vi "ADIS16448 IMU Example.vi"() -> ()   [LabVIEW 2018]
doc: "SimpleGyro Example\n\nThis example shows how to use a SimpleGyro sensor connected to the SPI port on the RoboRIO.\n\nThis example expects a USB cable connected from your development PC to the Type B USB Jack (next to the power input) on the roboRIO."
uses:
  ADIS16448 IMU/ADIS16448_IMU.lvlib
panel:
  out "Number of times failed":i32
  in  "Stahp":bool
  out "error out":errorcluster
  out "Z Angle":dbl
  in  "Calibrate On Open?":bool=TRUE
  out "IMU Angle Delta":cluster{"X":dbl, "Y":dbl, "Z":dbl} {"X" scale=-180.0..180.0; "Y" scale=-180.0..180.0; "Z" scale=-180.0..180.0}
  out "IMU AHRS":cluster{"Pitch":dbl, "Roll":dbl, "Yaw":dbl} {"Roll" scale=-180.0..180.0; "Pitch" scale=-90.0..90.0}
  out "IMU Data Out":T1 {"X Accel (g)" format="%#_3g"; "Y Accel (g)" format="%#_3g"; "Z Accel (g)" format="%#_3g"}
  in  "AHRS Algorithm":enum16{"Complementary", "Madgwick"}(ring)
  in  "AHRS Yaw Axis":enum16{"X", "Y", "Z"}(ring)=enum."Z"
  out "Sensor Ready?":bool
  out "IMU AHRS":cluster{"Pitch":dbl, "Roll":dbl, "Yaw":dbl}
  out "IMU Angle Delta":cluster{"X":dbl, "Y":dbl, "Z":dbl}
  in  "Reset Deltas?":bool
  out "Device Found?":bool
  in  "stop":bool
  # "FRC Analog Devices ADIS16448 IMU Example"
  # "Raw IMU Output Data"
  # "FRC ADI MXP Placement"
  # "Minimum LabVIEW version required: FRC 2019.0.0"
  # "Juan Chong -  Analog Devices Inc. - juan.chong@analog.com"
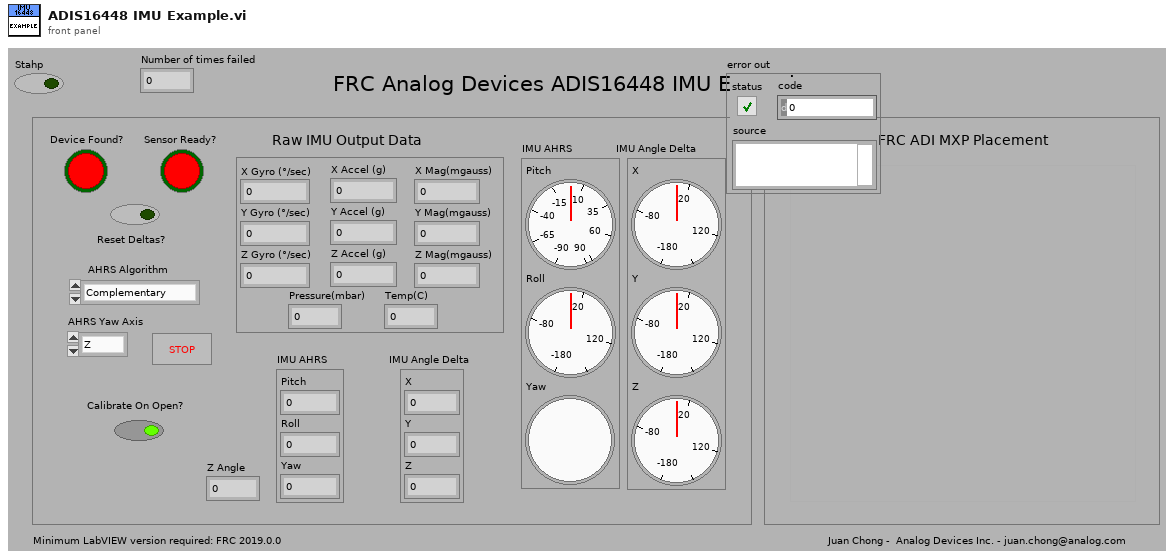
[diagram p1: front panel]
types:
  T1 = cluster{"X Gyro (°/sec)":dbl, "Y Gyro (°/sec)":dbl, "Z Gyro (°/sec)":dbl, "X Accel (g)":dbl, "Y Accel (g)":dbl, "Z Accel (g)":dbl, "X Mag(mgauss)":dbl, "Y Mag(mgauss)":dbl, "Z Mag(mgauss)":dbl, "Pressure(mbar)":dbl, "Temp(C)":dbl}
  T2 = typedef "ADIS16448_IMU.lvlib/ADI_IMU_ADIS16448_IMUDevRef.ctl" = cluster{"DevStatus":errorcluster, "Handle":i32, "SPI Bus":T3, "Device Found":bool, "Device Ready":bool, "Yaw Axis":enum16{"X", "Y", "Z"}, "AHRS Algorithm":enum16{"Complementary", "Madgwick"}, "Serial":u16, "Lot ID 2":u16, "Lot ID 1":u16, "Bytes Per Sample":u16, "Calibrate On Open?":bool}
  T3 = typedef "spi_bus.ctl" = enum16{"SPI On-Board, CS0", "SPI On-Board, CS1", "SPI On-Board, CS2", "SPI On-Board, CS3", "SPI MXP", "Invalid"}
  T4 = cluster{"X Angle":dbl, "Y Angle":dbl, "Z Angle":dbl}
  T5 = cluster{"X Gyro":dbl, "Y Gyro":dbl, "Z Gyro":dbl, "X Accel":dbl, "Y Accel":dbl, "Z Accel":dbl, "X Mag":dbl, "Y Mag":dbl, "Z Mag":dbl, "Pressure":dbl, "Temp":dbl}
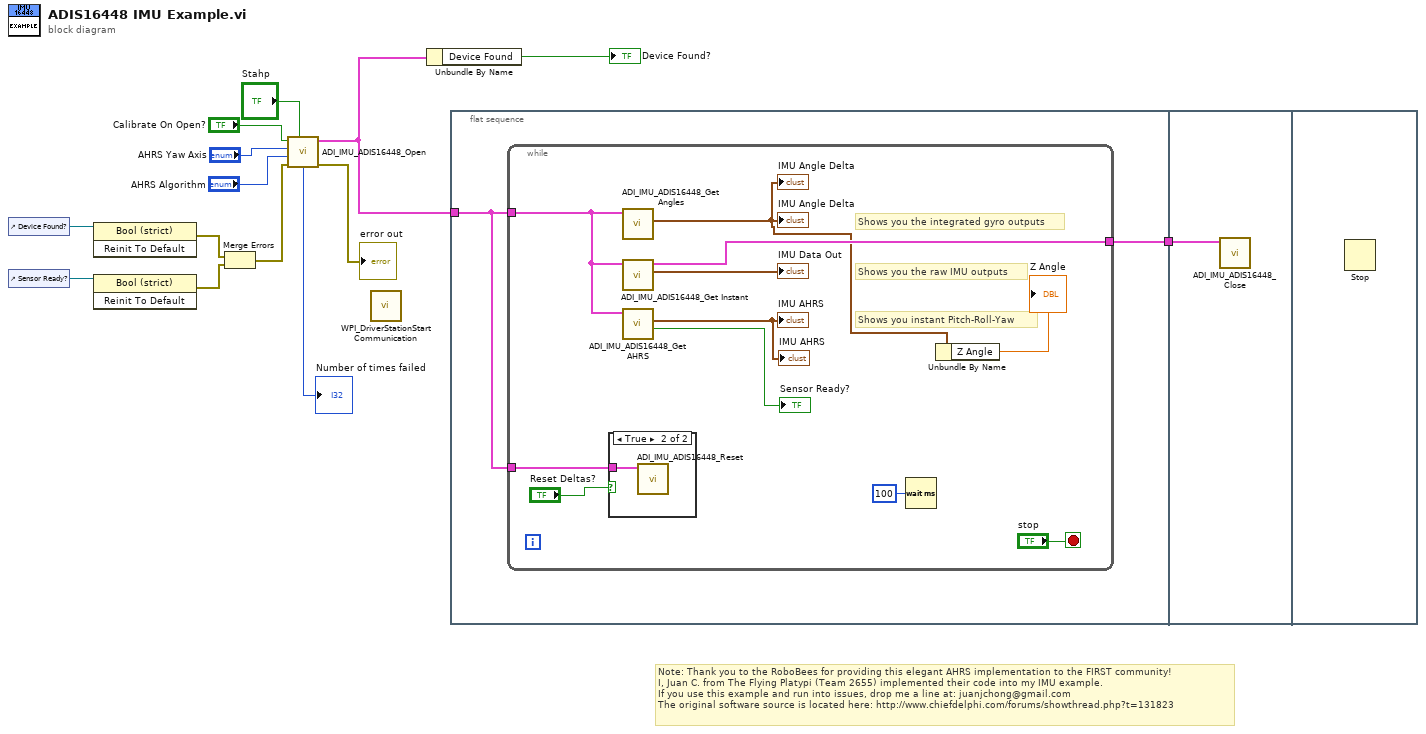
[diagram p0: block diagram]
diagram:
  # "Note: Thank you to the RoboBees for providing this elegant AHRS implementation to the FIRST community!\nI, Juan C. from The Flying Platypi (Team 2655) implemented their code into my IMU example.\nIf you use this example and run into issues, drop me a line at: juanjchong@gmail.com\nThe original software source is located here: http://www.chiefdelphi.com/forums/showthread.php?t=131823"
  n1 = control-ref of="Device Found?"() -> (w9:refnum<vi>)
  n2 = control-ref of="Sensor Ready?"() -> (w8:refnum<vi>)
  n3 = invoke class="Bool (strict)" method="Reinit To Default"(reference=w9) -> (error out=w7:errorcluster)  [unwired: 2 in, 2 out]
  n4 = invoke class="Bool (strict)" method="Reinit To Default"(reference=w8) -> (error out=w6:errorcluster)  [unwired: 2 in, 2 out]
  n5 = Merge Errors(w7, w6) -> (w5:errorcluster)
  n6 = call "ADI_IMU_ADIS16448_Open.vi"("Stahp"="Stahp", "error in"=w5, "AHRS Algorithm"="AHRS Algorithm", "Yaw Axis"="AHRS Yaw Axis", "Calibrate On Open"="Calibrate On Open?") -> ("error out"=→"error out":errorcluster, "ADI IMU DevRef Out"=w12:T2, "Number of times failed"=→"Number of times failed":i32)  [unwired: 4 in]
  n7 = call <vilib>:"WPI_DriverStationStart Communication.vi"() -> ()  [unwired: 12 in]
  n8 = Unbundle By Name(w12) -> ("Device Found"=→"Device Found?":bool)
  n9 = flat-sequence {
    tunnel: w12 -> [w16]
    tunnel: [w15] -> w11
    tunnel: w11 -> [w29]
    frame #0 {
      n10 = while {
        tunnel: w16 -> [w20]
        tunnel: w16 -> [w26]
        tunnel: [w21] -> w15
        stop <- "stop" stop-if-true
        # "Shows you the integrated gyro outputs"
        # "Shows you the raw IMU outputs"
        # "Shows you instant Pitch-Roll-Yaw"
        n11 = case shown="True" "Reset Deltas?" {
          tunnel: w26 -> [_ w28]
          frame False {
          }
          frame True {
            n12 = call "ADI_IMU_ADIS16448_Reset.vi"("ADI IMU DevRef"=w28) -> ()  [unwired: 9 in, 2 out]
          }
        }
        n13 = call "ADI_IMU_ADIS16448_Get Angles.vi"("ADI IMU DevRef"=w20) -> ("IMU Angles Out"=w18:T4)  [unwired: 7 in, 3 out]
        "IMU Angle Delta" <- w18
        "IMU Angle Delta" <- w18
        n14 = call "ADI_IMU_ADIS16448_Get Instant.vi"("ADI IMU DevRef"=w20) -> ("IMU Data Out"=→"IMU Data Out":T5, "ADI IMU DevRef Out"=w21:T2)  [unwired: 7 in, 2 out]
        n15 = call "ADI_IMU_ADIS16448_Get AHRS.vi"("ADI IMU DevRef"=w20) -> ("Sensor Ready Out"=→"Sensor Ready?":bool, "IMU AHRS Out"=→"IMU AHRS" →"IMU AHRS":cluster{"Pitch":dbl, "Roll":dbl, "Yaw":dbl})  [unwired: 7 in, 2 out]
        n16 = Wait (ms)(milliseconds to wait=u32 100) -> ()  [unwired: 1 out]
        n17 = Unbundle By Name(w18) -> ("Z Angle"=→"Z Angle":dbl)
      }
    }
    frame #1 {
      n18 = call "ADI_IMU_ADIS16448_Close.vi"("ADI IMU DevRef"=w29) -> ()  [unwired: 10 in, 1 out]
    }
    frame #2 {
      n19 = Stop() -> ()  [unwired: 1 in]
    }
  }
